vi "Dresden R2R Sputter 03.02.2018 IY24.vi"() -> ()   [LabVIEW 2009] (continued)
                          n13680 = Or(x=w20282, y=w20281) -> (x .or. y?=w20280:bool)
                        }
                      }
                      frame #1 {
                      }
                    }
                  }
                  frame #4 {
                    n13681 = local read "Semi"() -> (w20290:bool)
                    n13682 = case shown="False" w20290 {
                      frame #0 {
                        n13683 = local write "CH1_2trns_18"(TRUE ("CH1_2trns_7")) -> ()
                        n13684 = Wait (ms)(milliseconds to wait=u32 500) -> ()  [unwired: 1 out]
                      }
                      frame #1 {
                      }
                    }
                  }
                }
              }
              frame #1 {
              }
            }
          }
          frame #20 {
            n13685 = local read "Semi"() -> (w20293:bool)
            n13686 = case shown="False" w20293 {
              frame #0 {
                n13687 = local write "CH1_2trns_19"(TRUE ("CH1_2trns_18")) -> ()
                n13688 = local write "Cnt_Do_Buzzer"(TRUE ("Transfer_ch1_2")) -> ()
                n13689 = Wait (ms)(milliseconds to wait=u32 1500) -> ()  [unwired: 1 out]
              }
              frame #1 {
              }
            }
          }
          frame #21 {
            n13690 = local read "Semi"() -> (w20297:bool)
            n13691 = case shown="False" w20297 {
              frame #0 {
                n13692 = local write "ch_present_position"(2.0 ("ch_present_position")) -> ()
                n13693 = local write "Transfer_ch3_2"(FALSE ("Transfer_ch1_2")) -> ()
                n13694 = local write "Cnt_Do_Buzzer"(FALSE ("Transfer_ch1_2")) -> ()
                n13695 = Wait (ms)(milliseconds to wait=u32 500) -> ()  [unwired: 1 out]
              }
              frame #1 {
              }
            }
          }
        }
      }
      frame #5 {
        n13696 = stacked-sequence {
          frame #0 {
            n13697 = Wait (ms)(milliseconds to wait=u32 1500) -> ()  [unwired: 1 out]
            n13698 = local write "Clean_trnsfr_3_4"(TRUE ("Clean_trnsfr_1_2")) -> ()
            n13699 = local write "system_status"("Chamber 3 to Chamber 4 Transfer Process in Progress." ("system_status")) -> ()
            n13700 = local write "final_process_messages"("Chamber 3 to Chamber 4  Transfer Process was completed." ("final_process_messages")) -> ()
          }
          frame #1 {
            n13701 = stacked-sequence {
              frame #0 {
                n13702 = local write "Routine_check_transfer"(TRUE ("Routine_check_transfer")) -> ()
                n13703 = Wait (ms)(milliseconds to wait=u32 100) -> ()  [unwired: 1 out]
              }
              frame #1 {
                n13704 = while {
                  i -> [w20315]
                  stop <- w20311 stop-if-true
                  n13705 = Greater Or Equal?(x=w20315, y=1500) -> (x >= y?=w20312:bool)
                  n13706 = Wait Until Next ms Multiple(millisecond multiple=u32 200) -> ()  [unwired: 1 out]
                  n13707 = case shown="True" w20312 {
                    frame #0 {
                    }
                    frame #1 {
                      # "Hata mesajı"
                      n13708 = local write "Semi"(TRUE ("Semi")) -> ()
                    }
                  }
                  n13709 = local read "Routine_check_transfer"() -> (w20308:bool)
                  n13710 = local read "Semi"() -> (w20310:bool)
                  n13711 = Not(x=w20308) -> (.not. x?=w20309:bool)
                  n13712 = Or(x=w20309, y=w20310) -> (x .or. y?=w20311:bool)
                }
              }
              frame #2 {
                n13713 = Wait (ms)(milliseconds to wait=u32 500) -> ()  [unwired: 1 out]
              }
            }
          }
          frame #2 {
            # "STARTED UP CH3"
            n13714 = disable-structure shown="Disabled" {
              frame #0 {
                n13715 = local read "Semi"() -> (w20318:bool)
                n13716 = case shown="False" w20318 {
                  frame #0 {
                    n13717 = local read "started_up_ch3"() -> (w20319:bool)
                    n13718 = case shown="False" w20319 {
                      frame #0 {
                        n13719 = stacked-sequence {
                          frame #0 {
                            n13720 = local read "Semi"() -> (w20320:bool)
                            n13721 = case shown="False" w20320 {
                              frame #0 {
                                n13722 = local write "Start_up_ch3"(TRUE ("Start_up_ch2")) -> ()
                              }
                              frame #1 {
                              }
                            }
                          }
                          frame #1 {
                            n13723 = local read "Semi"() -> (w20322:bool)
                            n13724 = case shown="False" w20322 {
                              frame #0 {
                                n13725 = Wait (ms)(milliseconds to wait=u32 16000) -> ()  [unwired: 1 out]
                              }
                              frame #1 {
                              }
                            }
                          }
                          frame #2 {
                            n13726 = local read "Semi"() -> (w20324:bool)
                            n13727 = case shown="False" w20324 {
                              frame #0 {
                                n13728 = while {
                                i -> [w20329]
                                stop <- w20326 stop-if-true
                                n13729 = Greater?(x=w20329, y=80) -> (0:w20327:bool)
                                n13730 = local read "started_up_ch3"() -> (w20325:bool)
                                n13731 = case shown="True" w20327 {
                                frame #0 {
                                }
                                frame #1 {
                                n13732 = local write "Semi"(TRUE ("Semi")) -> ()
                                n13733 = local write "Error Message"("Chamber 1 Pressure is not suitable  \nfor transfer process!\nPlease check connections." ("Error Message")) -> ()
                                }
                                }
                                n13734 = case shown="False" w20325 {
                                tunnel: [FALSE TRUE] -> w20326
                                frame #0 {
                                n13735 = Wait Until Next ms Multiple(millisecond multiple=u32 200) -> ()  [unwired: 1 out]
                                }
                                frame #1 {
                                }
                                }
                                }
                              }
                              frame #1 {
                              }
                            }
                          }
                          frame #3 {
                            n13736 = local read "Semi"() -> (w20335:bool)
                            n13737 = case shown="False" w20335 {
                              frame #0 {
                                n13738 = local write "CH1_2_trns_0"(TRUE ("CH1_2_trns_0")) -> ()
                                n13739 = Wait (ms)(milliseconds to wait=u32 1000) -> ()  [unwired: 1 out]
                              }
                              frame #1 {
                              }
                            }
                          }
                        }
                      }
                      frame #1 {
                      }
                    }
                  }
                  frame #1 {
                  }
                }
              }
              frame #1 {
              }
            }
          }
          frame #3 {
            # "STARTED UP CH2"
            n13740 = disable-structure shown="Disabled" {
              frame #0 {
                n13741 = local read "Semi"() -> (w20338:bool)
                n13742 = case shown="False" w20338 {
                  frame #0 {
                    n13743 = local read "started_up_ch2"() -> (w20339:bool)
                    n13744 = case shown="False" w20339 {
                      frame #0 {
                        n13745 = stacked-sequence {
                          frame #0 {
                            n13746 = local read "Semi"() -> (w20340:bool)
                            n13747 = case shown="False" w20340 {
                              frame #0 {
                                n13748 = local write "Start_up_ch2"(TRUE ("Start_up_ch2")) -> ()
                              }
                              frame #1 {
                              }
                            }
                          }
                          frame #1 {
                            n13749 = local read "Semi"() -> (w20342:bool)
                            n13750 = case shown="False" w20342 {
                              frame #0 {
                                n13751 = Wait (ms)(milliseconds to wait=u32 18000) -> ()  [unwired: 1 out]
                              }
                              frame #1 {
                              }
                            }
                          }
                          frame #2 {
                            n13752 = local read "Semi"() -> (w20344:bool)
                            n13753 = case shown="False" w20344 {
                              frame #0 {
                                n13754 = while {
                                i -> [w20349]
                                stop <- w20346 stop-if-true
                                n13755 = Greater?(x=w20349, y=90) -> (0:w20347:bool)
                                n13756 = local read "started_up_ch2"() -> (w20345:bool)
                                n13757 = case shown="True" w20347 {
                                frame #0 {
                                }
                                frame #1 {
                                n13758 = local write "Semi"(TRUE ("Semi")) -> ()
                                n13759 = local write "Error Message"("Chamber 2 Pressure is not suitable  \nfor transfer process!\nPlease check connections." ("Error Message")) -> ()
                                }
                                }
                                n13760 = case shown="False" w20345 {
                                tunnel: [FALSE TRUE] -> w20346
                                frame #0 {
                                n13761 = Wait Until Next ms Multiple(millisecond multiple=u32 200) -> ()  [unwired: 1 out]
                                }
                                frame #1 {
                                }
                                }
                                }
                              }
                              frame #1 {
                              }
                            }
                          }
                          frame #3 {
                            n13762 = local read "Semi"() -> (w20355:bool)
                            n13763 = case shown="False" w20355 {
                              frame #0 {
                                n13764 = local write "CH1_2_trns_1"(TRUE ("CH1_2_trns_0")) -> ()
                                n13765 = Wait (ms)(milliseconds to wait=u32 1000) -> ()  [unwired: 1 out]
                              }
                              frame #1 {
                              }
                            }
                          }
                        }
                      }
                      frame #1 {
                      }
                    }
                  }
                  frame #1 {
                  }
                }
              }
              frame #1 {
              }
            }
          }
          frame #4 {
            # "TRNS GV-BP OPEN"
            n13766 = local read "Semi"() -> (w20358:bool)
            n13767 = case shown="False" w20358 {
              frame #0 {
                n13768 = stacked-sequence {
                  frame #0 {
                    n13769 = local read "Semi"() -> (w20359:bool)
                    n13770 = case shown="False" w20359 {
                      frame #0 {
                        n13771 = while {
                          i -> [w20366]
                          stop <- w20361 stop-if-true
                          n13772 = Greater?(x=w20366, y=50) -> (0:w20364:bool)
                          n13773 = local read "Ch3_Trns_gv_bp2_di"() -> (w20360:bool)
                          n13774 = case shown="True" w20364 {
                            frame #0 {
                            }
                            frame #1 {
                              n13775 = local write "Semi"(TRUE ("Semi")) -> ()
                              n13776 = local write "Error Message"("Transfer process was cancelled.\nPlease check CH1-Trns-GV connections." ("Error Message")) -> ()
                            }
                          }
                          n13777 = case shown="False" w20360 {
                            tunnel: [FALSE TRUE] -> w20363
                            frame #0 {
                              n13778 = Wait Until Next ms Multiple(millisecond multiple=u32 200) -> ()  [unwired: 1 out]
                              n13779 = local write "Ch3_Trns_gv_bp2_do"(TRUE ("Ch1_pet_cool_up_do")) -> ()
                            }
                            frame #1 {
                            }
                          }
                          n13780 = local read "Semi"() -> (w20362:bool)
                          n13781 = Or(x=w20363, y=w20362) -> (x .or. y?=w20361:bool)
                        }
                      }
                      frame #1 {
                      }
                    }
                  }
                  frame #1 {
                    n13782 = local read "Semi"() -> (w20373:bool)
                    n13783 = case shown="False" w20373 {
                      frame #0 {
                        n13784 = Wait (ms)(milliseconds to wait=u32 500) -> ()  [unwired: 1 out]
                      }
                      frame #1 {
                      }
                    }
                  }
                  frame #2 {
                    n13785 = local read "Semi"() -> (w20375:bool)
                    n13786 = case shown="False" w20375 {
                      frame #0 {
                        n13787 = while {
                          i -> [w20382]
                          stop <- w20377 stop-if-true
                          n13788 = Greater?(x=w20382, y=50) -> (0:w20380:bool)
                          n13789 = local read "Ch4_Trns_gv_bp_di"() -> (w20376:bool)
                          n13790 = case shown="True" w20380 {
                            frame #0 {
                            }
                            frame #1 {
                              n13791 = local write "Semi"(TRUE ("Semi")) -> ()
                              n13792 = local write "Error Message"("Transfer process was cancelled.\nPlease check CH1-Trns-GV connections." ("Error Message")) -> ()
                            }
                          }
                          n13793 = case shown="False" w20376 {
                            tunnel: [FALSE TRUE] -> w20379
                            frame #0 {
                              n13794 = local write "Ch4_Trns_gv_bp_do"(TRUE ("Ch1_pet_cool_up_do")) -> ()
                              n13795 = Wait Until Next ms Multiple(millisecond multiple=u32 200) -> ()  [unwired: 1 out]
                            }
                            frame #1 {
                            }
                          }
                          n13796 = local read "Semi"() -> (w20378:bool)
                          n13797 = Or(x=w20379, y=w20378) -> (x .or. y?=w20377:bool)
                        }
                      }
                      frame #1 {
                      }
                    }
                  }
                  frame #3 {
                    n13798 = local read "Semi"() -> (w20389:bool)
                    n13799 = case shown="False" w20389 {
                      frame #0 {
                        n13800 = Wait (ms)(milliseconds to wait=u32 500) -> ()  [unwired: 1 out]
                      }
                      frame #1 {
                      }
                    }
                  }
                }
              }
              frame #1 {
              }
            }
          }
          frame #5 {
            # "TRNS GV OPEN"
            n13801 = local read "Semi"() -> (w20391:bool)
            n13802 = case shown="False" w20391 {
              frame #0 {
                n13803 = stacked-sequence {
                  frame #0 {
                    n13804 = local read "Semi"() -> (w20392:bool)
                    n13805 = case shown="False" w20392 {
                      frame #0 {
                        n13806 = local write "Ch3_Trns_gv_close_do"(FALSE ("Ch1_pet_cool_up_do")) -> ()
                      }
                      frame #1 {
                      }
                    }
                  }
                  frame #1 {
                    n13807 = local read "Semi"() -> (w20394:bool)
                    n13808 = case shown="False" w20394 {
                      frame #0 {
                        n13809 = while {
                          i -> [w20401]
                          stop <- w20396 stop-if-true
                          n13810 = Greater?(x=w20401, y=500) -> (0:w20399:bool)
                          n13811 = local read "Ch3_Trns_gv_open_di"() -> (w20395:bool)
                          n13812 = case shown="True" w20399 {
                            frame #0 {
                            }
                            frame #1 {
                              n13813 = local write "Semi"(TRUE ("Semi")) -> ()
                              n13814 = local write "Error Message"("Transfer process was cancelled.\nPlease check CH1-Trns-GV connections." ("Error Message")) -> ()
                            }
                          }
                          n13815 = case shown="False" w20395 {
                            tunnel: [FALSE TRUE] -> w20398
                            frame #0 {
                              n13816 = Wait Until Next ms Multiple(millisecond multiple=u32 200) -> ()  [unwired: 1 out]
                              n13817 = local write "Ch3_Trns_gv_open_do"(TRUE ("Ch1_pet_cool_up_do")) -> ()
                            }
                            frame #1 {
                            }
                          }
                          n13818 = local read "Semi"() -> (w20397:bool)
                          n13819 = Or(x=w20398, y=w20397) -> (x .or. y?=w20396:bool)
                        }
                      }
                      frame #1 {
                      }
                    }
                  }
                  frame #2 {
                    n13820 = local read "Semi"() -> (w20408:bool)
                    n13821 = case shown="False" w20408 {
                      frame #0 {
                        n13822 = local write "CH1_2trns_2"(TRUE ("CH1_2trns_5")) -> ()
                        n13823 = Wait (ms)(milliseconds to wait=u32 500) -> ()  [unwired: 1 out]
                      }
                      frame #1 {
                      }
                    }
                  }
                }
              }
              frame #1 {
              }
            }
          }
          frame #6 {
            # "TRNS GV control Trnsgv 2_3"
            n13824 = local read "Semi"() -> (w20411:bool)
            n13825 = case shown="False" w20411 {
              frame #0 {
                n13826 = stacked-sequence {
                  frame #0 {
                    n13827 = local read "Semi"() -> (w20412:bool)
                    n13828 = case shown="False" w20412 {
                      frame #0 {
                        n13829 = while {
                          i -> [w20419]
                          stop <- w20414 stop-if-true
                          n13830 = Greater?(x=w20419, y=50) -> (0:w20417:bool)
                          n13831 = local read "Ch3_TGV_control_di"() -> (w20413:bool)
                          n13832 = case shown="True" w20417 {
                            frame #0 {
                            }
                            frame #1 {
                              n13833 = local write "Semi"(TRUE ("Semi")) -> ()
                              n13834 = local write "Error Message"("Transfer process was cancelled.\nPlease check TRNS-GV connections." ("Error Message")) -> ()
                            }
                          }
                          n13835 = case shown="True" w20413 {
                            tunnel: [TRUE FALSE] -> w20416
                            frame #0 {
                            }
                            frame #1 {
                              n13836 = Wait Until Next ms Multiple(millisecond multiple=u32 200) -> ()  [unwired: 1 out]
                              n13837 = local write "Ch3_TGV_control_do"(FALSE ("Ch1_pet_cool_up_do")) -> ()
                            }
                          }
                          n13838 = local read "Semi"() -> (w20415:bool)
                          n13839 = Or(x=w20416, y=w20415) -> (x .or. y?=w20414:bool)
                        }
                      }
                      frame #1 {
                      }
                    }
                  }
                  frame #1 {
                    n13840 = local read "Semi"() -> (w20426:bool)
                    n13841 = case shown="False" w20426 {
                      frame #0 {
                        n13842 = local write "CH1_2trns_3"(TRUE ("CH1_2trns_5")) -> ()
                        n13843 = Wait (ms)(milliseconds to wait=u32 500) -> ()  [unwired: 1 out]
                      }
                      frame #1 {
                      }
                    }
                  }
                }
              }
              frame #1 {
              }
            }
          }
          frame #7 {
            # "TRNS GV control Trnsgv 2_3"
            n13844 = local read "Semi"() -> (w20429:bool)
            n13845 = case shown="False" w20429 {
              frame #0 {
                n13846 = stacked-sequence {
                  frame #0 {
                    n13847 = local read "Semi"() -> (w20430:bool)
                    n13848 = case shown="False" w20430 {
                      frame #0 {
                        n13849 = while {
                          i -> [w20437]
                          stop <- w20432 stop-if-true
                          n13850 = Greater?(x=w20437, y=50) -> (0:w20435:bool)
                          n13851 = local read "Ch1_Trns_interlock_di"() -> (w20431:bool)
                          n13852 = case shown="True" w20435 {
                            frame #0 {
                            }
                            frame #1 {
                              n13853 = local write "Semi"(TRUE ("Semi")) -> ()
                              n13854 = local write "Error Message"("Transfer process was cancelled.\nPlease check TRNS-GV connections." ("Error Message")) -> ()
                            }
                          }
                          n13855 = case shown="False" w20431 {
                            tunnel: [w20439 TRUE] -> w20434
                            frame #0 {
                              n13856 = local read "Ch1_TGV_control_di"() -> (w20438:bool)
                              n13857 = case shown="False" w20438 {
                                tunnel: [FALSE TRUE] -> w20439
                                frame #0 {
                                n13858 = Wait Until Next ms Multiple(millisecond multiple=u32 200) -> ()  [unwired: 1 out]
                                n13859 = local write "Ch1_TGV_control_do"(TRUE ("Ch1_pet_cool_up_do")) -> ()
                                }
                                frame #1 {
                                }
                              }
                            }
                            frame #1 {
                            }
                          }
                          n13860 = local read "Semi"() -> (w20433:bool)
                          n13861 = Or(x=w20434, y=w20433) -> (x .or. y?=w20432:bool)
                        }
                      }
                      frame #1 {
                      }
                    }
                  }
                  frame #1 {
                    n13862 = local read "Semi"() -> (w20447:bool)
                    n13863 = case shown="False" w20447 {
                      frame #0 {
                        n13864 = local write "CH1_2trns_3"(TRUE ("CH1_2trns_5")) -> ()
                        n13865 = Wait (ms)(milliseconds to wait=u32 500) -> ()  [unwired: 1 out]
                      }
                      frame #1 {
                      }
                    }
                  }
                }
              }
              frame #1 {
              }
            }
          }
          frame #8 {
            # "TRNS GV control Trnsgv 3_4"
            n13866 = local read "Semi"() -> (w20450:bool)
            n13867 = case shown="False" w20450 {
              frame #0 {
                n13868 = stacked-sequence {
                  frame #0 {
                    n13869 = local read "Semi"() -> (w20451:bool)
                    n13870 = case shown="False" w20451 {
                      frame #0 {
                        n13871 = while {
                          i -> [w20458]
                          stop <- w20453 stop-if-true
                          n13872 = Greater?(x=w20458, y=50) -> (0:w20456:bool)
                          n13873 = local read "Ch2_Trns_interlock_di"() -> (w20452:bool)
                          n13874 = case shown="True" w20456 {
                            frame #0 {
                            }
                            frame #1 {
                              n13875 = local write "Semi"(TRUE ("Semi")) -> ()
                              n13876 = local write "Error Message"("Transfer process was cancelled.\nPlease check TRNS-GV connections." ("Error Message")) -> ()
                            }
                          }
                          n13877 = case shown="False" w20452 {
                            tunnel: [w20460 TRUE] -> w20455
                            frame #0 {
                              n13878 = local read "Ch2_TGV_control_di"() -> (w20459:bool)
                              n13879 = case shown="False" w20459 {
                                tunnel: [FALSE TRUE] -> w20460
                                frame #0 {
                                n13880 = Wait Until Next ms Multiple(millisecond multiple=u32 200) -> ()  [unwired: 1 out]
                                n13881 = local write "Ch2_TGV_control_do"(TRUE ("Ch1_pet_cool_up_do")) -> ()
                                }
                                frame #1 {
                                }
                              }
                            }
                            frame #1 {
                            }
                          }
                          n13882 = local read "Semi"() -> (w20454:bool)
                          n13883 = Or(x=w20455, y=w20454) -> (x .or. y?=w20453:bool)
                        }
                      }
                      frame #1 {
                      }
                    }
                  }
                  frame #1 {
                    n13884 = local read "Semi"() -> (w20468:bool)
                    n13885 = case shown="False" w20468 {
                      frame #0 {
                        n13886 = local write "CH1_2trns_4"(TRUE ("CH1_2trns_5")) -> ()
                        n13887 = Wait (ms)(milliseconds to wait=u32 500) -> ()  [unwired: 1 out]
                      }
                      frame #1 {
                      }
                    }
                  }
                }
              }
              frame #1 {
              }
            }
          }
          frame #9 {
            # "Right slow deactive"
            n13888 = local read "Semi"() -> (w20471:bool)
            n13889 = case shown="False" w20471 {
              frame #0 {
                n13890 = stacked-sequence {
                  frame #0 {
                    n13891 = local read "Semi"() -> (w20472:bool)
                    n13892 = case shown="False" w20472 {
                      frame #0 {
                        n13893 = while {
                          i -> [w20475]
                          stop <- w20476 stop-if-true
                          n13894 = Greater?(x=w20475, y=50) -> (0:w20473:bool)
                          n13895 = local read "Cnt_Right_slow_di"() -> (w20479:bool)
                          n13896 = case shown="True" w20473 {
                            frame #0 {
                            }
                            frame #1 {
                              n13897 = local write "Semi"(TRUE ("Semi")) -> ()
                              n13898 = local write "Error Message"("Transfer process was\ncancelled.Please check right slow sensor." ("Error Message")) -> ()
                            }
                          }
                          n13899 = case shown="False" w20479 {
                            tunnel: [FALSE ("Ch1_pet_cool_up_do") TRUE ("Ch1_pet_cool_up_do")] -> w20478
                            frame #0 {
                              n13900 = Wait Until Next ms Multiple(millisecond multiple=u32 200) -> ()  [unwired: 1 out]
                              n13901 = local write "Cnt_Right_slow_do"(TRUE ("Ch1_pet_cool_up_do")) -> ()
                            }
                            frame #1 {
                            }
                          }
                          n13902 = local read "Semi"() -> (w20477:bool)
                          n13903 = Or(x=w20478, y=w20477) -> (x .or. y?=w20476:bool)
                        }
                      }
                      frame #1 {
                      }
                    }
                  }
                  frame #1 {
                    n13904 = local read "Semi"() -> (w20486:bool)
                    n13905 = case shown="False" w20486 {
                      frame #0 {
                        n13906 = local write "CH1_2trns_5"(TRUE ("CH1_2trns_7")) -> ()
                        n13907 = Wait (ms)(milliseconds to wait=u32 500) -> ()  [unwired: 1 out]
                      }
                      frame #1 {
                      }
                    }
                  }
                }
              }
              frame #1 {
              }
            }
          }
          frame #10 {
            # "Right limit deactive"
            n13908 = local read "Semi"() -> (w20489:bool)
            n13909 = case shown="False" w20489 {
              frame #0 {
                n13910 = stacked-sequence {
                  frame #0 {
                    n13911 = local read "Semi"() -> (w20490:bool)
                    n13912 = case shown="False" w20490 {
                      frame #0 {
                        n13913 = while {
                          i -> [w20491]
                          stop <- w20495 stop-if-true
                          n13914 = Greater?(x=w20491, y=50) -> (0:w20493:bool)
                          n13915 = local read "Cnt_Right_limit_di"() -> (w20497:bool)
                          n13916 = case shown="True" w20493 {
                            frame #0 {
                            }
                            frame #1 {
                              n13917 = local write "Semi"(TRUE ("Semi")) -> ()
                              n13918 = local write "Error Message"("Transfer process was\ncancelled.Please check right limit sensor." ("Error Message")) -> ()
                            }
                          }
                          n13919 = case shown="False" w20497 {
                            tunnel: [FALSE ("Ch1_pet_cool_up_do") TRUE ("Ch1_pet_cool_up_do")] -> w20496
                            frame #0 {
                              n13920 = Wait Until Next ms Multiple(millisecond multiple=u32 200) -> ()  [unwired: 1 out]
                              n13921 = local write "Cnt_Right_limit_do"(TRUE ("Ch1_pet_cool_up_do")) -> ()
                            }
                            frame #1 {
                            }
                          }
                          n13922 = local read "Semi"() -> (w20494:bool)
                          n13923 = Or(x=w20496, y=w20494) -> (x .or. y?=w20495:bool)
                        }
                      }
                      frame #1 {
                      }
                    }
                  }
                  frame #1 {
                    n13924 = local read "Semi"() -> (w20504:bool)
                    n13925 = case shown="False" w20504 {
                      frame #0 {
                        n13926 = local write "CH1_2trns_6"(TRUE ("CH1_2trns_7")) -> ()
                        n13927 = Wait (ms)(milliseconds to wait=u32 500) -> ()  [unwired: 1 out]
                      }
                      frame #1 {
                      }
                    }
                  }
                }
              }
              frame #1 {
              }
            }
          }
          frame #11 {
            # "Left slow deactive"
            n13928 = local read "Semi"() -> (w20507:bool)
            n13929 = case shown="False" w20507 {
              frame #0 {
                n13930 = stacked-sequence {
                  frame #0 {
                    n13931 = local read "Semi"() -> (w20508:bool)
                    n13932 = case shown="False" w20508 {
                      frame #0 {
                        n13933 = while {
                          i -> [w20509]
                          stop <- w20513 stop-if-true
                          n13934 = Greater?(x=w20509, y=50) -> (0:w20511:bool)
                          n13935 = local read "Cnt_Left_slow_di"() -> (w20515:bool)
                          n13936 = case shown="True" w20511 {
                            frame #0 {
                            }
                            frame #1 {
                              n13937 = local write "Semi"(TRUE ("Semi")) -> ()
                              n13938 = local write "Error Message"("Transfer process was\ncancelled.Please check left slow sensor." ("Error Message")) -> ()
                            }
                          }
                          n13939 = case shown="False" w20515 {
                            tunnel: [FALSE ("Ch1_pet_cool_up_do") TRUE ("Ch1_pet_cool_up_do")] -> w20514
                            frame #0 {
                              n13940 = Wait Until Next ms Multiple(millisecond multiple=u32 200) -> ()  [unwired: 1 out]
                              n13941 = local write "Cnt_Left_slow_do"(TRUE ("Ch1_pet_cool_up_do")) -> ()
                            }
                            frame #1 {
                            }
                          }
                          n13942 = local read "Semi"() -> (w20512:bool)
                          n13943 = Or(x=w20514, y=w20512) -> (x .or. y?=w20513:bool)
                        }
                      }
                      frame #1 {
                      }
                    }
                  }
                  frame #1 {
                    n13944 = local read "Semi"() -> (w20522:bool)
                    n13945 = case shown="False" w20522 {
                      frame #0 {
                        n13946 = local write "CH1_2trns_7"(TRUE ("CH1_2trns_6b")) -> ()
                        n13947 = Wait (ms)(milliseconds to wait=u32 500) -> ()  [unwired: 1 out]
                      }
                      frame #1 {
                      }
                    }
                  }
                }
              }
              frame #1 {
              }
            }
          }
          frame #12 {
            # "Left limit deactive"
            n13948 = local read "Semi"() -> (w20525:bool)
            n13949 = case shown="False" w20525 {
              frame #0 {
                n13950 = stacked-sequence {
                  frame #0 {
                    n13951 = local read "Semi"() -> (w20526:bool)
                    n13952 = case shown="False" w20526 {
                      frame #0 {
                        n13953 = while {
                          i -> [w20527]
                          stop <- w20531 stop-if-true
                          n13954 = Greater?(x=w20527, y=50) -> (0:w20529:bool)
                          n13955 = local read "Cnt_Left_limit_di"() -> (w20533:bool)
                          n13956 = case shown="True" w20529 {
                            frame #0 {
                            }
                            frame #1 {
                              n13957 = local write "Semi"(TRUE ("Semi")) -> ()
                              n13958 = local write "Error Message"("Transfer process was\ncancelled.Please check left limit sensor." ("Error Message")) -> ()
                            }
                          }
                          n13959 = case shown="False" w20533 {
                            tunnel: [FALSE ("Ch1_pet_cool_up_do") TRUE ("Ch1_pet_cool_up_do")] -> w20532
                            frame #0 {
                              n13960 = Wait Until Next ms Multiple(millisecond multiple=u32 200) -> ()  [unwired: 1 out]
                              n13961 = local write "Cnt_Left_limit_do"(TRUE ("Ch1_pet_cool_up_do")) -> ()
                            }
                            frame #1 {
                            }
                          }
                          n13962 = local read "Semi"() -> (w20530:bool)
                          n13963 = Or(x=w20532, y=w20530) -> (x .or. y?=w20531:bool)
                        }
                      }
                      frame #1 {
                      }
                    }
                  }
                  frame #1 {
                    n13964 = local read "Semi"() -> (w20540:bool)
                    n13965 = case shown="False" w20540 {
                      frame #0 {
                        n13966 = local write "CH1_2trns_8"(TRUE ("CH1_2trns_6c")) -> ()
                        n13967 = Wait (ms)(milliseconds to wait=u32 500) -> ()  [unwired: 1 out]
                      }
                      frame #1 {
                      }
                    }
                  }
                }
              }
              frame #1 {
              }
            }
          }
          frame #13 {
            # "Casette Direction"
            n13968 = local read "Semi"() -> (w20543:bool)
            n13969 = case shown="False" w20543 {
              frame #0 {
                n13970 = stacked-sequence {
                  frame #0 {
                    n13971 = local read "Semi"() -> (w20544:bool)
                    n13972 = case shown="False" w20544 {
                      frame #0 {
                        n13973 = while {
                          i -> [w20550]
                          stop <- w20545 stop-if-true
                          n13974 = Greater?(x=w20550, y=50) -> (0:w20551:bool)
                          n13975 = case shown="True" w20551 {
                            frame #0 {
                            }
                            frame #1 {
                              n13976 = local write "Semi"(TRUE ("Semi")) -> ()
                              n13977 = local write "Error Message"("Transfer process was cancelled.\nPlease check Casette Direction connections." ("Error Message")) -> ()
                            }
                          }
                          n13978 = local read "Casette_servo_left_direction_di"() -> (w20548:bool)
                          n13979 = case shown="False" w20548 {
                            tunnel: [FALSE ("Casette_servo_left_direction_do") TRUE ("Casette_servo_left_direction_do")] -> w20547
                            frame #0 {
                              n13980 = Wait Until Next ms Multiple(millisecond multiple=u32 200) -> ()  [unwired: 1 out]
                              n13981 = local write "Casette_servo_left_direction_do"(TRUE ("Casette_servo_left_direction_do")) -> ()
                            }
                            frame #1 {
                            }
                          }
                          n13982 = local read "Semi"() -> (w20546:bool)
                          n13983 = Or(x=w20547, y=w20546) -> (x .or. y?=w20545:bool)
                        }
                      }
                      frame #1 {
                      }
                    }
                  }
                  frame #1 {
                    n13984 = local read "Semi"() -> (w20558:bool)
                    n13985 = case shown="False" w20558 {
                      frame #0 {
                        n13986 = local write "CH1_2trns_9"(TRUE ("CH1_2trns_7")) -> ()
                        n13987 = Wait (ms)(milliseconds to wait=u32 500) -> ()  [unwired: 1 out]
                      }
                      frame #1 {
                      }
                    }
                  }
                }
              }
              frame #1 {
              }
            }
          }
          frame #14 {
            # "SET CASSETTE SERVO  SPEED 300"
            n13988 = local read "Semi"() -> (w20561:bool)
            n13989 = case shown="False" w20561 {
              frame #0 {
                n13990 = stacked-sequence {
                  frame #0 {
                    n13991 = local read "Semi"() -> (w20562:bool)
                    n13992 = case shown="False" w20562 {
                      frame #0 {
                        n13993 = local write "Cassette_servo_speed_value"(u16 300 ("Cassette_servo_speed_value")) -> ()
                      }
                      frame #1 {
                      }
                    }
                  }
                  frame #1 {
                    n13994 = local read "Semi"() -> (w20564:bool)
                    n13995 = case shown="False" w20564 {
                      frame #0 {
                        n13996 = Wait (ms)(milliseconds to wait=u32 200) -> ()  [unwired: 1 out]
                      }
                      frame #1 {
                      }
                    }
                  }
                  frame #2 {
                    n13997 = local read "Semi"() -> (w20566:bool)
                    n13998 = case shown="False" w20566 {
                      frame #0 {
                        n13999 = local write "Cassette_servo_speed_auto_set"(TRUE ("Cassette_servo_speed_set")) -> ()
                      }
                      frame #1 {
                      }
                    }
                  }
                  frame #3 {
                    n14000 = local read "Semi"() -> (w20568:bool)
                    n14001 = case shown="False" w20568 {
                      frame #0 {
                        n14002 = Wait (ms)(milliseconds to wait=u32 200) -> ()  [unwired: 1 out]
                      }
                      frame #1 {
                      }
                    }
                  }
                  frame #4 {
                    n14003 = local read "Semi"() -> (w20570:bool)
                    n14004 = case shown="False" w20570 {
                      frame #0 {
                        n14005 = local write "CH1_2trns_10"(TRUE ("CH1_2trns_7")) -> ()
                        n14006 = Wait (ms)(milliseconds to wait=u32 500) -> ()  [unwired: 1 out]
                      }
                      frame #1 {
                      }
                    }
                  }
                }
              }
              frame #1 {
              }
            }
          }
          frame #15 {
            # "Casette Servo Start"
            n14007 = local read "Semi"() -> (w20573:bool)
            n14008 = case shown="False" w20573 {
              frame #0 {
                n14009 = stacked-sequence {
                  frame #0 {
                    n14010 = while {
                      i -> [w20579]
                      stop <- w20574 stop-if-true
                      n14011 = Greater?(x=w20579, y=50) -> (0:w20580:bool)
                      n14012 = local read "Casette_servo_start/stop_di"() -> (w20577:bool)
                      n14013 = case shown="True" w20580 {
                        frame #0 {
                        }
                        frame #1 {
                          n14014 = local write "Semi"(TRUE ("Semi")) -> ()
                          n14015 = local write "Error Message"("Transfer process was cancelled.\nPlease check Casette connections." ("Error Message")) -> ()
                        }
                      }